vi "MPS_main.vi"() -> ()   [LabVIEW 2021] (continued)
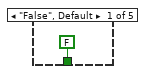
[diagram p2: hidden frame]
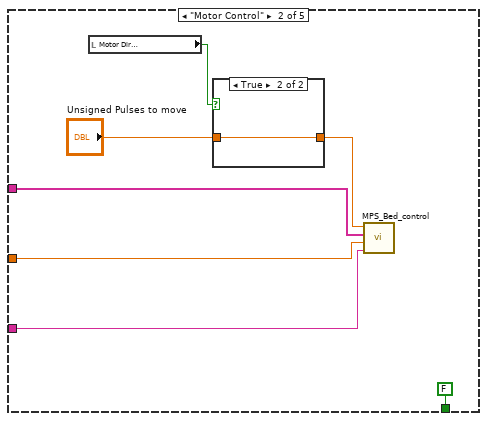
[diagram p3: hidden frame]
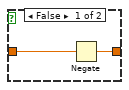
[diagram p4: hidden frame]
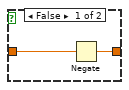
[diagram p5: hidden frame]
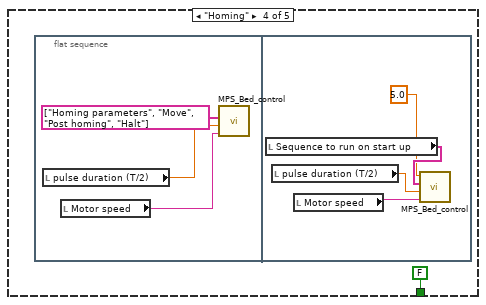
[diagram p6: hidden frame]
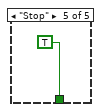
[diagram p7: hidden frame]
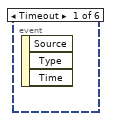
[diagram p8: hidden frame]
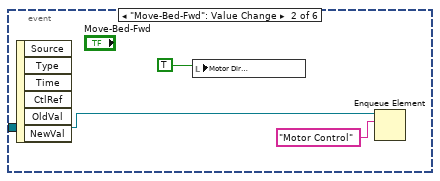
[diagram p9: hidden frame]
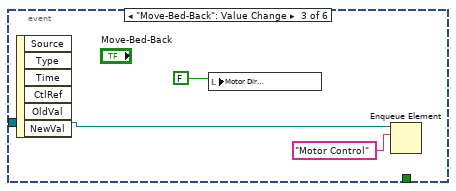
[diagram p10: hidden frame]
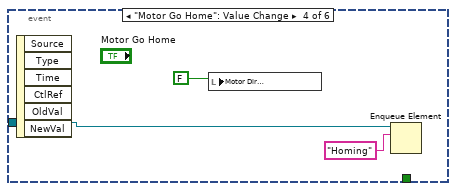
[diagram p11: hidden frame]
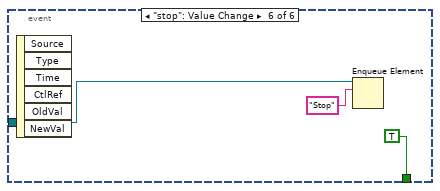
[diagram p12: hidden frame]
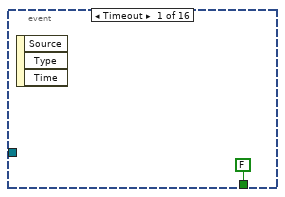
[diagram p13: hidden frame]
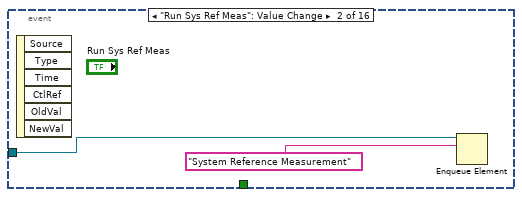
[diagram p14: hidden frame]
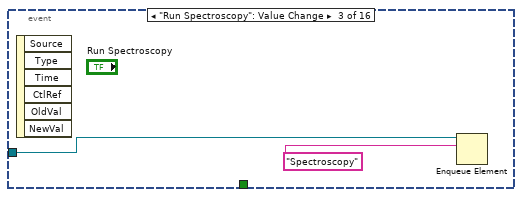
[diagram p15: hidden frame]
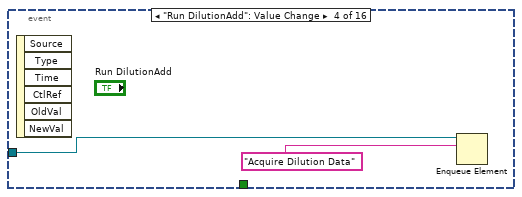
[diagram p16: hidden frame]
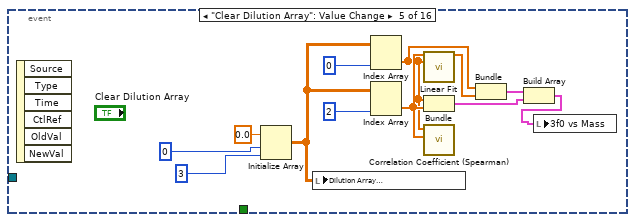
[diagram p17: hidden frame]
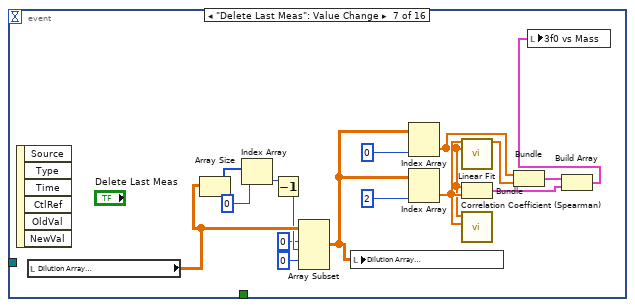
[diagram p18: hidden frame]
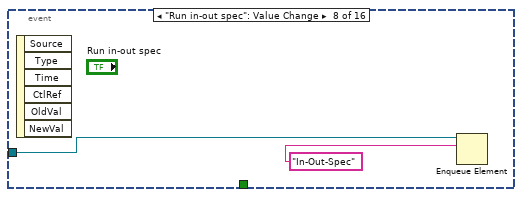
[diagram p19: hidden frame]
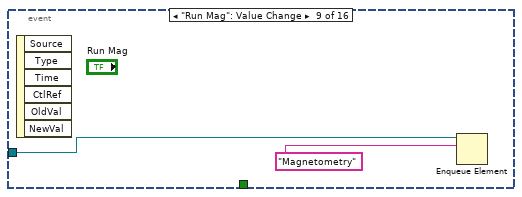
[diagram p20: hidden frame]
        n162 = Index Array(array=w205, index (col)=0 ("disabled index (col)")) -> (element=w206:dbl[])  [unwired: 1 in]
        n163 = call <vilib>:"Std Deviation and Variance.vi"("X"=w212) -> ("mean"=→"mean3f0":dbl, "standard deviation"=→"standard deviation 3f0":dbl)  [unwired: 1 in, 1 out]
        n164 = call <vilib>:"Std Deviation and Variance.vi"("X"=w206) -> ("mean"=→"meanf0":dbl, "standard deviation"=→"standard deviation f0":dbl)  [unwired: 1 in, 1 out]
        n165 = local read "Pulses From Home to Max Sig"() -> (w199:dbl)
        n166 = case shown="True" "Save Spectroscopy" {
          tunnel: w225 -> [_ w253]
          tunnel: w224 -> [_ w252]
          tunnel: w205 -> [_ w248]
          tunnel: w215 -> [_ w247]
          tunnel: w214 -> [_ w246]
          tunnel: w213 -> [_ w245]
          tunnel: w203 -> [_ w244]
          tunnel: w202 -> [_ w243]
          tunnel: w201 -> [_ w242]
          tunnel: w200 -> [_ w240]
          tunnel: w199 -> [_ w236]
          frame False {
          }
          frame True {
            w229 = u16 0 items=["Spec.", "Mag.", "In Out Spec"] ("Ring")
            n167 = local read "Sample MetaData Cluster"() -> (w230:T1)
            n168 = local read "name identifier"() -> (w231:string)
            n169 = local read "Study and Experiment Description"() -> (w234:T5)
            n170 = local read "Sample MetaData Cluster"() -> (w233:T1)
            n171 = Initialize Array(0.0 ("element"), 1 ("dimension size")) -> (w237:dbl[])
            n172 = local read "Base path"() -> (w232:path)
            n173 = call "Spectrometer_File_Naming.vi"("Description"=w231, "Sample MetaData Cluster"=w230, "Ring"=w229) -> ("Output Name"=w228:string)  [unwired: 8 in]
            n174 = Bundle By Name(cluster=T8 {"Drive IMon"=array[500000 elements], "Rx Time Domain"=array[500000 elements], "Rx Empty Bore"=array[500000 elements], "BMon"=array[500000 elements], "Bias IMon"=array[500000 elements], "TF-Corr-MagOverTime"=[], "Interpolated Rx TF-Mag"=[], "Interpolated Rx TF-Phase"=[]} ("Time Domain Cluster"), "Drive IMon"=w246, "Rx Time Domain"=w245, "Rx Empty Bore"=w253, "BMon"=w252, "Bias IMon"=w237, "TF-Corr-MagOverTime"=w244, "Interpolated Rx TF-Mag"=w243, "Interpolated Rx TF-Phase"=w240) -> (w254:T8)
            n175 = local read "Scanner Description"() -> (w235:T4)
            n176 = call "file_path.vi"("name identifier"=w228, "Base path"=w232) -> ("HDF path"=w250:path)  [unwired: 7 in, 2 out]
            n177 = global read "MPS_global_variables.vi" "TxRx_Params"() -> (w249:T2)
            n178 = local write "Recent File Name"(w228) -> ()
            n179 = call "save_MPS_spectroscopy_hdf.vi"("file path"=w250, "Device Name"=tag "H1", "Phase Rx over time"=w247, "Mag Rx over time"=w248, "TxRx_Params"=w249, "Rx_f0-f8 Units"=w242, "Time Domain Cluster"=w254, "Sample MetaData Cluster"=w233, "Study and Experiment Description"=w234, "Scanner Description"=w235, "Points from home to max"=w236) -> ()  [unwired: 5 in]
          }
        }
      }
      frame "Acquire Dilution Data" {
        n180 = Enqueue Element(queue=w325, element="Idle") -> ()  [unwired: 2 in, 3 out]
        n181 = Initialize Array(0.0 ("element"), 0 ("dimension size"), 9 ("dimension size")) -> (w322:dbl[][])
        n182 = while {
          shift-right: [w336] -> w317
          shift-left: w322 -> [w337]
          i -> [w335]
          stop <- w328 stop-if-true
          n183 = local read "RxEmptyBore-Spec"() -> (w334:dbl[])
          n184 = call "MPS_Spectroscopy_Core.vi"("EmptyBoreBaseline_Spec"=w334, "ms delay"="ms delay 2", "Spec samples\nto crop"="Spec samples\nto crop 3") -> ("mag f1-f9"=w331:dbl[], "Expected mT Spec Drive"=→"Expected mT Spec Drive 3":dbl, "THD"=→"THD 2":dbl)  [unwired: 2 in, 12 out]
          n185 = Insert Into Array(array=w337, index (row)=w335, new element=w331) -> (w336:dbl[][])  [unwired: 1 in]
          n186 = Greater Or Equal?(x=w335, y="Num Dil Series Runs") -> (x >= y?=w328:bool)
        }
        n187 = local read "Dilution Array\nConc,f0,f3"() -> (w315:dbl[][])
        n188 = local read "Sample MetaData Cluster"() -> (w310:T1)
        n189 = Index Array(array=w317, index (col)=2 ("index")) -> (element=w320:dbl[])  [unwired: 1 in]
        n190 = Index Array(array=w317, index (col)=0 ("disabled index (col)")) -> (element=w318:dbl[])  [unwired: 1 in]
        n191 = call <vilib>:"Std Deviation and Variance.vi"("X"=w318) -> ("mean"=w302:dbl)  [unwired: 1 in, 2 out]
        n192 = call <vilib>:"Std Deviation and Variance.vi"("X"=w320) -> ("mean"=w303:dbl)  [unwired: 1 in, 2 out]
        n193 = Unbundle By Name(w310) -> ("Sample Mass (ug)"=w311:dbl)
        n194 = Array Size(array=w315) -> (size(s)=w314:i32[])
        n195 = Index Array(array=w314, index=0) -> (element=w313:i32)
        n196 = Build Array(w311, w302, w303) -> (w309:dbl[])
        n197 = Bundle By Name(cluster=T9 {"slope min"=-inf, "slope max"=inf, "intercept min"=-inf, "intercept max"=inf} ("parameter bounds"), "intercept min"=0.0) -> (w295:T9)
        n198 = Insert Into Array(array=w315, index (row)=w313, new element=w309) -> (w307:dbl[][])  [unwired: 1 in]
        n199 = local write "Dilution Array\nConc,f0,f3"(w307) -> ()
        n200 = Index Array(array=w307, index (col)=0 ("disabled index (col)")) -> (element=w301:dbl[])  [unwired: 1 in]
        n201 = Index Array(array=w307, index (col)=2 ("disabled index (col)")) -> (element=w299:dbl[])  [unwired: 1 in]
        n202 = call <vilib>:"Linear Fit.vi"("Y"=w299, "X"=w301, "parameter bounds"=w295) -> ("Best Linear Fit"=w305:dbl[])  [unwired: 8 in, 4 out]
        n203 = call <vilib>:"Correlation Coefficient.vi"("Y"=w299, "X"=w301) -> ("r^2"=→"r^2":dbl)  [unwired: 8 in, 1 out]
        n204 = Bundle("Dilution Array\nConc,f0,f3"=w301, "Dilution Array\nConc,f0,f3"=w299) -> (w298:T13)  [unwired: 1 in]
        n205 = Bundle("Dilution Array\nConc,f0,f3"=w301, "Best Linear Fit"=w305) -> (w297:T14)  [unwired: 1 in]
        n206 = Build Array(w297, w298) -> (→"3f0 vs Mass":T6)
      }
      frame "In-Out-Spec" {
        w375 = 0
        n207 = Enqueue Element(queue=w393, element="Idle") -> ()  [unwired: 2 in, 3 out]
        n208 = Initialize Array(0.0 ("element"), 9 ("dimension size"), 1 ("dimension size")) -> (w376:dbl[][])
        n209 = Initialize Array(0.0 ("element"), 9 ("dimension size"), 1 ("dimension size")) -> (w377:dbl[][])
        n210 = Initialize Array(0.0 ("element"), 1 ("dimension size")) -> (w361:dbl[])
        n211 = Multiply(x="Number of cycles", y=2) -> (x*y=w365:i32)
        n212 = flat-sequence {
          tunnel: w377 -> [w404]
          tunnel: w376 -> [w403]
          tunnel: w375 -> [w402]
          tunnel: w365 -> [w399]
          tunnel: w361 -> [w398]
          tunnel: cluster{"f0":dbl, "df":dbl, "magnitude":dbl[]} {"f0"=0.0, "df"=49.55401387512537, "magnitude"=array[10090 elements]} ("Rx FFT 3") -> [w396]
          tunnel: [w401] -> w350
          tunnel: [w400] -> w349
          tunnel: [w397] -> w348
          tunnel: [w395] -> w347
          tunnel: [w498] -> w355
          tunnel: [w499] -> w360
          tunnel: [w500] -> w370
          tunnel: [w501] -> w374
          tunnel: w350 -> [w501]
          tunnel: w349 -> [w500]
          tunnel: w348 -> [w499]
          tunnel: w347 -> [w498]
          tunnel: [w495] -> w346
          tunnel: [w494] -> w345
          tunnel: [w493] -> w344
          frame #0 {
            n213 = for {
              N: w399 -> [_]
              shift-right: [w421] -> w400
              shift-left: w404 -> [w423]
              shift-right: [w420] -> w401
              shift-left: w403 -> [w422]
              tunnel: w402 -> [_]
              shift-right: [w411] -> w397
              shift-left: w398 -> [w412]
              shift-right: [w405] -> w395
              shift-left: w396 -> [_]
              i -> [w419]
              n214 = flat-sequence {
                tunnel: w423 -> [w433]
                tunnel: w422 -> [w432]
                tunnel: [w431] -> w416
                tunnel: [w430] -> w415
                tunnel: w414 -> [w429]
                tunnel: w412 -> [w428]
                tunnel: w407 -> [w427]
                tunnel: [w426] -> w410
                tunnel: [w425] -> w406
                tunnel: [w424] -> w405
                tunnel: [w488] -> w420
                tunnel: [w489] -> w421
                tunnel: w416 -> [w489]
                tunnel: w415 -> [w488]
                tunnel: w413 -> [w483]
                tunnel: [w473] -> w411
                tunnel: w410 -> [w473]
                tunnel: w406 -> [_]
                frame #0 {
                  n215 = while {
                    shift-right: [w470] -> w431
                    shift-left: w433 -> [w471]
                    shift-right: [w465] -> w430
                    shift-left: w432 -> [w469]
                    tunnel: w429 -> [w447]
                    tunnel: w427 -> [w441]
                    shift-right: [w440] -> w426
                    shift-left: w428 -> [w443]
                    tunnel: [w436] -> w425
                    tunnel: [w435] -> w424
                    i -> [w450]
                    stop <- w466 stop-if-true
                    w459 = T11 1 items=["Rectangle"=0, "Hanning"=1, "Hamming"=2, "Blackman-Harris"=3, "Exact Blackman"=4, "Blackman"=5, "Flat Top"=6, "4 Term B-Harris "=7, "7 Term B-Harris"=8, "Low Sidelobe"=9, "Blackman Nuttall"=11, "Triangle"=30, "Bartlett-Hanning"=31, "Bohman"=32, "Parzen"=33, "Welch"=34, "Kaiser"=60, "Dolph-Chebyshev"=61, "Gaussian"=62] ("window")
                    n216 = local read "RxEmptyBore-Spec"() -> (w464:dbl[])
                    n217 = local write "Bed moving"(FALSE ("Bed moving")) -> ()
                    n218 = local read "Run number"() -> (w451:i32)
                    n219 = Greater Or Equal?(x=w450, y="Num acq per\ncycle") -> (x >= y?=w466:bool)
                    n220 = Increment(x=w451) -> (x+1=w442:i32)
                    n221 = call "MPS_Spectroscopy_Core.vi"("EmptyBoreBaseline_Spec"=w464, "ms delay"="ms delay\nevery Spec", "Spec samples\nto crop"="Spec samples\nto crop_InOut") -> ("Raw Measured"=w444:dbl[], "f0 Complex"=w454:cdb, "phase f1-f9"=w467:dbl[], "TF Corr Rx FFT Mag"=→"Rx FFT 2":cluster{"f0":dbl, "df":dbl, "magnitude":dbl[]}, "Spec Waveform Baseline Sub"=w458:waveform(dbl), "3f0 Complex"=w457:cdb, "mag f1-f9"=w452:dbl[], "Expected mT Spec Drive"=→"Expected mT Spec Drive 2":dbl, "TF Corrected\nMagnetization over time"=w439:waveform(dbl)[], "Spec Time Domain"=→"Spec Time Domain 2":dbl[][], "THD"=→"Drive Imon THD 2":dbl)  [unwired: 2 in, 4 out]
                    n222 = Equal?(x=w450, y=0) -> (x = y?=w446:bool)
                    n223 = local write "Run number"(w442) -> ()
                    n224 = And(x=w446, y=w447) -> (x .and. y?=w448:bool)
                    n225 = Insert Into Array(array=w471, index (col)=w442, new element=w452) -> (w470:dbl[][])  [unwired: 1 in]
                    n226 = Insert Into Array(array=w469, index (col)=w442, new element=w467) -> (w465:dbl[][])  [unwired: 1 in]
                    n227 = Complex To Polar(r * e^(i*theta)=w454) -> (r=→"f0 over time 2":dbl)  [unwired: 1 out]
                    n228 = Complex To Polar(r * e^(i*theta)=w457) -> (r=→"3f0 over time 2":dbl)  [unwired: 1 out]
                    n229 = case shown="True" w448 {
                      tunnel: w444 -> [_ w472]
                      frame False {
                      }
                      frame True {
                        n230 = local write "RxEmptyBore-Spec"(w472) -> ()
                      }
                    }
                    n231 = Insert Into Array(array=w443, index=w442, new element=w441) -> (w440:dbl[])
                    n232 = Index Array(array=w439, index=1) -> (element=w437:waveform(dbl))
                    n233 = call-poly <vilib>:"FFT Spectrum (Mag-Phase).vi"("window"=w459, "time signal"=w458) -> ("magnitude"=w435:cluster{"f0":dbl, "df":dbl, "magnitude":dbl[]})  [unwired: 5 in, 4 out]
                    n234 = Unbundle By Name(w437) -> ("Y"=w436:dbl[])
                    "Loop Num 2" <- w450
                  }
                }
                frame #1 {
                  w480 = 0.0005 ("pulse duration (T/2)")
                  n235 = case shown="True" w483 {
                    tunnel: [w490 w491] -> w487
                    tunnel: "Pulses in/out" -> [w490 w492]
                    frame False {
                    }
                    frame True {
                      n236 = Negate(x=w492) -> (-x=w491:dbl)
                    }
                  }
                  n237 = local write "Bed moving"(TRUE) -> ()
                  n238 = Multiply(x="Pulses in/out", y=w480) -> (x*y=w482:dbl)
                  n239 = Multiply(x=w482, y=16.0) -> (x*y=w479:dbl)
                  n240 = Multiply(x=w479, y=1.25) -> (x*y=w477:dbl)
                  n241 = call "MPS_Bed_control.vi"("Motor speed"="Sixteenth step", "pulse duration (T/2)"=w480, "Sequence to run on start up"=string[] ["Move", "Halt"] ("Sequence to run on start up\n 2"), "Signed pulses to move"=w487) -> ()  [unwired: 8 in]
                  n242 = Multiply(x=1000.0, y=w477) -> (x*y=w475:dbl)
                  n243 = Wait (ms)(milliseconds to wait=w475) -> ()  [unwired: 1 out]
                }
              }
              n244 = Quotient & Remainder(x=w419, y=2) -> (x-y*floor(x/y)=w409:i32)  [unwired: 1 out]
              n245 = Decrement(x=w409) -> (x-1=w408:i32)
              n246 = Equal?(x=w409, y=0) -> (x = y?=w413:bool)
              n247 = Absolute Value(x=w408) -> (abs(x)=w407:i32)
              n248 = Not(x=w413) -> (.not. x?=w414:bool)
            }
          }
          frame #1 {
            # "Final Acq.\nwith sample in\nto save time domain"
            n249 = local read "Spec samples\nto crop_InOut"() -> (w496:dbl)
            n250 = local read "RxEmptyBore-Spec"() -> (w497:dbl[])
            n251 = call "MPS_Spectroscopy_Core.vi"("EmptyBoreBaseline_Spec"=w497, "Spec samples\nto crop"=w496) -> ("Spec Waveform Baseline Sub"=w495:waveform(dbl), "Drive IMon"=w494:waveform(dbl), "TF Corrected\nMagnetization over time"=w493:waveform(dbl)[])  [unwired: 3 in, 12 out]
          }
        }
        n252 = Unbundle By Name(w346) -> ("Y"=w341:dbl[])
        n253 = Unbundle By Name(w345) -> ("Y"=w340:dbl[])
        n254 = Array Subset(array=w370, index (row)=0 ("index"), index (col)=1 ("index")) -> (w369:dbl[][])  [unwired: 2 in]
        n255 = Array Subset(array=w374, index (row)=0 ("index"), index (col)=1 ("index")) -> (w373:dbl[][])  [unwired: 2 in]
        n256 = Array Subset(array=w360, index=1) -> (w358:dbl[])  [unwired: 1 in]
        n257 = Index Array(array=w344, index=1) -> (element=w342:waveform(dbl))
        n258 = Unbundle By Name(w342) -> ("Y"=w339:dbl[])
        n259 = local read "Study and Experiment Description"() -> (w386:T5)
        n260 = local read "Sample MetaData Cluster"() -> (w385:T1)
        n261 = local read "Empty Bore-BMon-Spec"() -> (w389:dbl[])
        n262 = global read "MPS_global_variables.vi" "Rx TF File"() -> (w354:string)
        n263 = local read "Scanner Description"() -> (w387:T4)
        n264 = local read "RxEmptyBore-Spec"() -> (w388:dbl[])
        n265 = call "get_freq_vector.vi"("FFT magnitude"=w355) -> ("Freq array"=w357:dbl[])  [unwired: 10 in]
        n266 = call "loadTF_resample.vi"("desired freqs"=w357, "mat file name"=w354) -> ("TF units from loaded file"=w351:string, "output TF phase"=w352:dbl[], "output TF mag"=w353:dbl[])  [unwired: 7 in]
        n267 = Initialize Array(0.0 ("element"), 1 ("dimension size")) -> (w390:dbl[])
        n268 = local read "Pulses From Home to Max Sig"() -> (w338:dbl)
        n269 = case shown="True" "Save Spectroscopy 2" {
          tunnel: w388 -> [_ w527]
          tunnel: w389 -> [_ w526]
          tunnel: w385 -> [_ w525]
          tunnel: w386 -> [_ w524]
          tunnel: w387 -> [_ w523]
          tunnel: w390 -> [_ w516]
          tunnel: w369 -> [_ w518]
          tunnel: w373 -> [_ w519]
          tunnel: w358 -> [_ w517]
          tunnel: w353 -> [_ w515]
          tunnel: w352 -> [_ w513]
          tunnel: w351 -> [_ w512]
          tunnel: w341 -> [_ w511]
          tunnel: w340 -> [_ w510]
          tunnel: w339 -> [_ w509]
          tunnel: w338 -> [_ w507]
          frame False {
          }
          frame True {
            w503 = u16 2 items=["Spec.", "Mag.", "In Out Spec"] ("Ring")
            n270 = local read "Sample MetaData Cluster"() -> (w505:T1)
            n271 = Bundle By Name(cluster=T8 {"Drive IMon"=array[500000 elements], "Rx Time Domain"=array[500000 elements], "Rx Empty Bore"=array[500000 elements], "BMon"=array[500000 elements], "Bias IMon"=array[500000 elements], "TF-Corr-MagOverTime"=[], "Interpolated Rx TF-Mag"=[], "Interpolated Rx TF-Phase"=[]} ("Time Domain Cluster 2"), "Drive IMon"=w510, "Rx Time Domain"=w511, "Rx Empty Bore"=w527, "BMon"=w526, "Bias IMon"=w516, "TF-Corr-MagOverTime"=w509, "Interpolated Rx TF-Mag"=w515, "Interpolated Rx TF-Phase"=w513) -> (w508:T8)
            n272 = local read "Base path"() -> (w504:path)
            n273 = local read "name identifier"() -> (w506:string)
            n274 = call "Spectrometer_File_Naming.vi"("Description"=w506, "Sample MetaData Cluster"=w505, "Ring"=w503) -> ("Output Name"=w502:string)  [unwired: 8 in]
            n275 = global read "MPS_global_variables.vi" "TxRx_Params"() -> (w520:T2)
            n276 = call "file_path.vi"("name identifier"=w502, "Base path"=w504) -> ("HDF path"=w521:path)  [unwired: 7 in, 2 out]
            n277 = local write "Recent File Name"(w502) -> ()
            n278 = call "save_MPS_spectroscopy_hdf.vi"("file path"=w521, "Device Name"=tag "H1", "Phase Rx over time"=w519, "Mag Rx over time"=w518, "TxRx_Params"=w520, "Rx_f0-f8 Units"=w512, "Time Domain Cluster"=w508, "Sample MetaData Cluster"=w525, "Study and Experiment Description"=w524, "Sample in_vs_Out"=w517, "Scanner Description"=w523, "Points from home to max"=w507) -> ()  [unwired: 4 in]
          }
        }
        "Run number" <- w375
      }
      frame "Update Meta" {
      }
      frame "Magnetometry" {
        w551 = T11 1 items=["Rectangle"=0, "Hanning"=1, "Hamming"=2, "Blackman-Harris"=3, "Exact Blackman"=4, "Blackman"=5, "Flat Top"=6, "4 Term B-Harris "=7, "7 Term B-Harris"=8, "Low Sidelobe"=9, "Blackman Nuttall"=11, "Triangle"=30, "Bartlett-Hanning"=31, "Bohman"=32, "Parzen"=33, "Welch"=34, "Kaiser"=60, "Dolph-Chebyshev"=61, "Gaussian"=62] ("window")
        n279 = Enqueue Element(queue=w560, element="Idle") -> ()  [unwired: 2 in, 3 out]
        n280 = local read "EmptyBoreBaseline_Mag"() -> (w542:dbl[])
        n281 = Array Size(array=w542) -> (size(s)=w538:i32)
        n282 = Initialize Array(0.0 ("element"), w538) -> (w537:dbl[])
        n283 = Initialize Array(0.0 ("element"), w538, "Num Mag Avgs") -> (w543:dbl[][])
        n284 = Multiply(x="Num Mag Avgs", y=2) -> (x*y=w532:i32)
        n285 = for {
          N: w532 -> [_]
          tunnel: [w582] -> w530
          tunnel: [w581] -> w552
          tunnel: [w580] -> w535
          shift-right: [w578] -> w540
          shift-left: w543 -> [w579]
          i -> [w572]
          n286 = Quotient & Remainder(x=w572, y=2) -> (x-y*floor(x/y)=w575:i32, floor(x/y)=w571:i32)
          n287 = flat-sequence {
            tunnel: [w597] -> w582
            tunnel: [w584] -> w580
            tunnel: w579 -> [w590]
            tunnel: [w595] -> w577
            tunnel: [w588] -> w576
            tunnel: w567 -> [w591]
            tunnel: w571 -> [w587]
            tunnel: w577 -> [w622]
            tunnel: w576 -> [w621]
            tunnel: w570 -> [w613]
            tunnel: [w622] -> w569
            tunnel: [w621] -> w568
            tunnel: [w627] -> w578
            tunnel: [w628] -> w581
            tunnel: w569 -> [w628]
            tunnel: w568 -> [w627]
            frame #0 {
              n288 = local read "EmptyBoreBaseline_Mag_BMon"() -> (w599:dbl[])
              n289 = local read "EmptyBoreBaseline_Mag"() -> (w600:dbl[])
              n290 = local write "Bed moving"(FALSE) -> ()
              n291 = call "MPS_Mag_Core.vi"("EmptyBoreBaseline_Mag_BMon"=w599, "EmptyBoreBaseline_Mag"=w600) -> ("Samples Per Acquisition"=w593:dbl, "Drive IMon"=w596:waveform(dbl), "Susceptibility Curves"=→"Susceptibility Curves":cluster{"Y":dbl[], "Y":dbl[]}[], "Rx Smooth"=→"Rx Smooth":dbl[], "Bias Current"=w597:waveform(dbl), "Rx_Raw"=w585:waveform(dbl), "RxBaselineSub"=w584:waveform(dbl))  [unwired: 5 in, 2 out]
              n292 = local write "Samples Per Acquisition"(w593) -> ()
              n293 = Unbundle By Name(w596) -> ("Y"=w595:dbl[])
              n294 = call "MPS_Mag_Proc_Spectrogram.vi"("Signal"=w584) -> ("Sensitivity profile"=→"Sensitivity profile":dbl[][])  [unwired: 9 in, 1 out]
              n295 = Unbundle By Name(w584) -> ("Y"=w583:dbl[])
              n296 = Unbundle By Name(w585) -> ("Y"=w589:dbl[])
              n297 = case shown="False" w591 {
                tunnel: w590 -> [w604 w606]
                tunnel: w589 -> [_ w605]
                tunnel: [w603 w606] -> w588
                tunnel: w587 -> [w602 _]
                tunnel: w583 -> [w601 _]
                frame False {
                  n298 = Replace Array Subset(array=w604, new element=w601, index (col)=w602) -> (w603:dbl[][])  [unwired: 1 in]
                  "RunNum" <- w602
                }
                frame True {
                  n299 = local write "EmptyBoreBaseline_Mag"(w605) -> ()
                }
              }
            }
            frame #1 {
              w611 = 0.0005 ("pulse duration (T/2)")
              n300 = case shown="True" w613 {
                tunnel: [w623 w624] -> w615
                tunnel: "Pulses in/out 2" -> [w623 w625]
                frame False {
                }
                frame True {
                  n301 = Negate(x=w625) -> (-x=w624:dbl)
                }
              }
              n302 = local write "Bed moving"(TRUE) -> ()
              n303 = Multiply(x="Pulses in/out 2", y=w611) -> (x*y=w616:dbl)
              n304 = Multiply(x=w616, y=16.0) -> (x*y=w617:dbl)
              n305 = Multiply(x=w617, y=1.25) -> (x*y=w618:dbl)
              n306 = call "MPS_Bed_control.vi"("Motor speed"="Sixteenth step", "pulse duration (T/2)"=w611, "Sequence to run on start up"=string[] ["Move", "Halt"] ("Sequence to run on start up\n 2"), "Signed pulses to move"=w615) -> ()  [unwired: 8 in]
              n307 = Multiply(x=1000.0, y=w618) -> (x*y=w619:dbl)
              n308 = Wait (ms)(milliseconds to wait=w619) -> ()  [unwired: 1 out]
            }
            frame #2 {
              n309 = Wait (ms)(milliseconds to wait="ms delay each run") -> ()  [unwired: 1 out]
            }
          }
          n310 = Equal?(x=w575, y=0) -> (x = y?=w570:bool)
          n311 = Not(x=w570) -> (.not. x?=w567:bool)
          "Sample Out" <- w567
          "Numeric" <- w572
        }
        n312 = for {
          N: "Num Mag Avgs" -> [_]
          shift-right: [w563] -> w536
          shift-left: w537 -> [w564]
          shift-right: [w562] -> _
          shift-left: w540 -> [w562]
          i -> [w566]
          n313 = Index Array(array=w562, index (col)=w566) -> (element=w565:dbl[])  [unwired: 1 in]
          n314 = Add(x=w565, y=w564) -> (x+y=w563:dbl[])
        }
        n315 = call-poly <vilib>:"FFT Spectrum (Mag-Phase).vi"("window"=w551, "time signal"=w535) -> ("magnitude"=w549:cluster{"f0":dbl, "df":dbl, "magnitude":dbl[]})  [unwired: 5 in, 4 out]
        n316 = global read "MPS_global_variables.vi" "Rx TF File"() -> (w548:string)
        n317 = Unbundle By Name(w530) -> ("Y"=w553:dbl[])
        n318 = call "get_freq_vector.vi"("FFT magnitude"=w549) -> ("Freq array"=w550:dbl[])  [unwired: 10 in]
        n319 = call "loadTF_resample.vi"("desired freqs"=w550, "mat file name"=w548) -> ("TF units from loaded file"=w545:string, "output TF phase"=w547:dbl[], "output TF mag"=w546:dbl[])  [unwired: 7 in]
        n320 = local read "Study and Experiment Description"() -> (w556:T5)
        n321 = local read "EmptyBoreBaseline_Mag_BMon"() -> (w558:dbl[])
        n322 = Divide(x=w536, y="Num Mag Avgs") -> (x/y=w531:dbl[])
        n323 = local read "Sample MetaData Cluster"() -> (w557:T1)
        n324 = local read "Scanner Description"() -> (w555:T4)
        n325 = local read "EmptyBoreBaseline_Mag"() -> (w559:dbl[])
        n326 = Bundle By Name(cluster=w530, "Y"=w531) -> (w529:waveform(dbl))
        n327 = call "MPS_Mag_Proc_Spectrogram.vi"("Signal"=w529) -> ("Sensitivity profile"=→"Sensitivity profile 2":dbl[][])  [unwired: 9 in, 1 out]
        n328 = local read "Pulses From Home to Max Sig"() -> (w544:dbl)
        n329 = case shown="True" "Save Mag data" {
          tunnel: w558 -> [_ w653]
          tunnel: w557 -> [_ w652]
          tunnel: w556 -> [_ w651]
          tunnel: w555 -> [_ w650]
          tunnel: w559 -> [_ w647]
          tunnel: w553 -> [_ w643]
          tunnel: w552 -> [_ w642]
          tunnel: w547 -> [_ w640]
          tunnel: w546 -> [_ w639]
          tunnel: w545 -> [_ w638]
          tunnel: w544 -> [_ w635]
          tunnel: w531 -> [_ w629]
          frame False {
          }
          frame True {
            w632 = u16 1 items=["Spec.", "Mag.", "In Out Spec"] ("Ring")
            n330 = local read "Sample MetaData Cluster"() -> (w634:T1)
            n331 = Bundle By Name(cluster=T8 {"Drive IMon"=array[500000 elements], "Rx Time Domain"=array[500000 elements], "Rx Empty Bore"=array[500000 elements], "BMon"=array[500000 elements], "Bias IMon"=array[500000 elements], "TF-Corr-MagOverTime"=[], "Interpolated Rx TF-Mag"=[], "Interpolated Rx TF-Phase"=[]} ("Time Domain Cluster 3"), "Drive IMon"=w642, "Rx Time Domain"=w629, "Rx Empty Bore"=w647, "BMon"=w653, "Bias IMon"=w643, "TF-Corr-MagOverTime"=dbl[] [], "Interpolated Rx TF-Mag"=w639, "Interpolated Rx TF-Phase"=w640) -> (w637:T8)
            n332 = local read "name identifier"() -> (w633:string)
            n333 = local read "Base path"() -> (w631:path)
            n334 = call "Spectrometer_File_Naming.vi"("Description"=w633, "Sample MetaData Cluster"=w634, "Ring"=w632) -> ("Output Name"=w630:string)  [unwired: 8 in]
            n335 = global read "MPS_global_variables.vi" "TxRx_Params"() -> (w645:T2)
            n336 = call "file_path.vi"("name identifier"=w630, "Base path"=w631) -> ("HDF path"=w648:path)  [unwired: 7 in, 2 out]
            n337 = Initialize Array(0.0 ("element")) -> (w644:dbl[][])  [unwired: 2 in]
            n338 = call "save_MPS_spectroscopy_hdf.vi"("file path"=w648, "Device Name"=tag "H1", "Phase Rx over time"=w644, "Mag Rx over time"=w644, "TxRx_Params"=w645, "Rx_f0-f8 Units"=w638, "Time Domain Cluster"=w637, "Sample MetaData Cluster"=w652, "Study and Experiment Description"=w651, "Scanner Description"=w650, "Points from home to max"=w635) -> ()  [unwired: 5 in]
            n339 = local write "Recent File Name"(w630) -> ()
          }
        }
      }
      frame "Acquire Empty Bore" {
        n340 = Enqueue Element(queue=w654, element="Idle") -> ()  [unwired: 2 in, 3 out]
        n341 = stacked-sequence {
          frame #0 {
            # "Data queue"
            # "Data queue"
            n342 = global read "MPS_global_variables.vi" "TxRx_Params"() -> (w665:T2)
            n343 = Unbundle By Name(w665) -> ("Tx cycles\nSpectroscopy"=w661:dbl, "sample rate"=w664:dbl, "Tx freq"=w663:dbl)
            n344 = Obtain Queue(element data type=waveform(dbl) {"t0"=timestamp(0 s since 1904-01-01), "dt"=1.0, "Y"=[]} ("Waveform")) -> (queue out=w666:refnum<queue>)  [unwired: 4 in, 2 out]
            n345 = Obtain Queue(element data type=waveform(dbl) {"t0"=timestamp(0 s since 1904-01-01), "dt"=1.0, "Y"=[]} ("Waveform")) -> (queue out=w658:refnum<queue>)  [unwired: 4 in, 2 out]
            n346 = Divide(x=w664, y=w663) -> (x/y=w662:dbl)
            n347 = Multiply(x=w661, y=w662) -> (x*y=w660:dbl)
            n348 = flat-sequence {
              tunnel: w666 -> [w668]
              tunnel: w660 -> [w671]
              tunnel: [w670] -> w659
              tunnel: w659 -> [w691]
              tunnel: w658 -> [w678]
              frame #0 {
                w673 = T11 1 items=["Rectangle"=0, "Hanning"=1, "Hamming"=2, "Blackman-Harris"=3, "Exact Blackman"=4, "Blackman"=5, "Flat Top"=6, "4 Term B-Harris "=7, "7 Term B-Harris"=8, "Low Sidelobe"=9, "Blackman Nuttall"=11, "Triangle"=30, "Bartlett-Hanning"=31, "Bohman"=32, "Parzen"=33, "Welch"=34, "Kaiser"=60, "Dolph-Chebyshev"=61, "Gaussian"=62] ("window")
                n349 = call <extravilib>:"Write.vi"("element"=1 ("number of readouts")) -> ("channel"=w676:T12)  [unwired: 1 out]
                n350 = Dequeue Element(queue=w668) -> (element=w667:waveform(dbl))  [unwired: 2 in, 3 out]
                n351 = Round To Nearest(number=w671) -> (nearest integer value=w670:dbl)
                n352 = Unbundle By Name(w667) -> ("Y"=w674:dbl[])
                "EmptyBoreBaseline_Spec" <- w674
                "RxEmptyBore-Spec" <- w674
                n353 = call-poly <vilib>:"FFT Spectrum (Mag-Phase).vi"("window"=w673, "time signal"=w667) -> ("magnitude"=w672:cluster{"f0":dbl, "df":dbl, "magnitude":dbl[]})  [unwired: 5 in, 4 out]
                n354 = call "MPS_transmit_receive.vi"("samples per readout"=w670, "Use Bias?"=FALSE, "InputChans"=enum16{"Rx", "BiasIMon", "TxIMon", "BMon"}."Rx", "channel input for max readouts"=w676, "Measurement Queue"=w668) -> ()  [unwired: 7 in]
                n355 = local write "Samples Per Acquisition"(w670) -> ()
                n356 = local write "EmptyBoreBaseline_Spec"(w674) -> ()
                n357 = Complex To Polar(r * e^(i*theta)=w672) -> ()  [unwired: 2 out]
              }
              frame #1 {
                n358 = Dequeue Element(queue=w678) -> (element=w680:waveform(dbl))  [unwired: 2 in, 3 out]
                n359 = Round To Nearest(number=w691) -> (nearest integer value=w694:dbl)
                n360 = call <extravilib>:"Write.vi"("element"=1 ("number of readouts")) -> ("channel"=w695:T12)  [unwired: 1 out]
                n361 = call "MPS_transmit_receive.vi"("samples per readout"=w694, "Use Bias?"=TRUE, "InputChans"=enum16{"Rx", "BiasIMon", "TxIMon", "BMon"}."BMon", "channel input for max readouts"=w695, "Measurement Queue"=w678) -> ()  [unwired: 7 in]
                n362 = call-poly <vilib>:"Mean.vi"("X"=w680) -> ("mean"=w690:dbl)  [unwired: 1 out]
                n363 = Subtract(x=w680, y=w690) -> (x-y=w688:waveform(dbl))
                n364 = Unbundle By Name(w680) -> ("Y"=→"Empty Bore-BMon-Spec":dbl[], "dt"=w687:dbl)
                n365 = call <vilib>:"Integral x(t).vi"("dt"=w687, "Initial Condition"=dbl[] [0.0], "X"=w688) -> ("Integral X"=w686:dbl[])  [unwired: 7 in, 1 out]
                n366 = Bundle By Name(cluster=w680, "Y"=w686) -> (w682:waveform(dbl))
                n367 = call-poly <vilib>:"Extract Single Tone Information.vi"("export mode"=T10."detected signal", "time signal in"=w682) -> ("exported signals"=w684:T15)  [unwired: 4 in, 5 out]
                n368 = Unbundle By Name(w684) -> ("exported time signal"=w683:waveform(dbl))
                n369 = Unbundle By Name(w683) -> ()  [unwired: 1 out]
              }
            }
          }
          frame #1 {
            n370 = Wait (ms)(milliseconds to wait=u32 100) -> ()  [unwired: 1 out]
          }
          frame #2 {
            # "Data queue"
            # "Data queue"
            n371 = global read "MPS_global_variables.vi" "TxRx_Params"() -> (w706:T2)
            n372 = Unbundle By Name(w706) -> ("Bias Periods\nMagnetometry"=w702:dbl, "sample rate"=w705:dbl, "Bias freq"=w704:dbl)
            n373 = Obtain Queue(element data type=waveform(dbl) {"t0"=timestamp(0 s since 1904-01-01), "dt"=1.0, "Y"=[]} ("Waveform")) -> (queue out=w707:refnum<queue>)  [unwired: 4 in, 2 out]
            n374 = Obtain Queue(element data type=waveform(dbl) {"t0"=timestamp(0 s since 1904-01-01), "dt"=1.0, "Y"=[]} ("Waveform")) -> (queue out=w700:refnum<queue>)  [unwired: 4 in, 2 out]
            n375 = Divide(x=w705, y=w704) -> (x/y=w703:dbl)
            n376 = Multiply(x=w702, y=w703) -> (x*y=w701:dbl)
            n377 = flat-sequence {
              tunnel: w707 -> [w709]
              tunnel: w701 -> [w712]
              tunnel: [w712] -> w699
              tunnel: w700 -> [w718]
              tunnel: w699 -> [w720]
              frame #0 {
                n378 = Dequeue Element(queue=w709) -> (element=w710:waveform(dbl))  [unwired: 2 in, 3 out]
                "RxEmptyBore-Mag" <- w710
                n379 = Round To Nearest(number=w712) -> (nearest integer value=w714:dbl)
                n380 = call <extravilib>:"Write.vi"("element"=1 ("number of readouts")) -> ("channel"=w715:T12)  [unwired: 1 out]
                n381 = Unbundle By Name(w710) -> ("Y"=w711:dbl[])
                "EmptyBoreBaseline_Mag" <- w711
                n382 = call "MPS_transmit_receive.vi"("samples per readout"=w714, "Use Bias?"=TRUE, "InputChans"=enum16{"Rx", "BiasIMon", "TxIMon", "BMon"}."Rx", "channel input for max readouts"=w715, "Measurement Queue"=w709) -> ()  [unwired: 7 in]
                n383 = local write "Samples Per Acquisition"(w714) -> ()
                n384 = local write "EmptyBoreBaseline_Mag"(w711) -> ()
              }
              frame #1 {
                (unwired) FALSE ("T=DriveMon \nF=BMon")
                n385 = call <extravilib>:"Write.vi"("element"=1 ("number of readouts")) -> ("channel"=w722:T12)  [unwired: 1 out]
                n386 = Dequeue Element(queue=w718) -> (element=w719:waveform(dbl))  [unwired: 2 in, 3 out]
                n387 = Round To Nearest(number=w720) -> (nearest integer value=w723:dbl)
                n388 = Unbundle By Name(w719) -> ("Y"=w724:dbl[])
                "EmptyBoreBaseline_Mag_BMon" <- w724
                n389 = call "MPS_transmit_receive.vi"("samples per readout"=w723, "Use Bias?"=TRUE, "InputChans"=enum16{"Rx", "BiasIMon", "TxIMon", "BMon"}."BMon", "channel input for max readouts"=w722, "Measurement Queue"=w718) -> ()  [unwired: 7 in]
                n390 = local write "Samples Per Acquisition"(w723) -> ()
                n391 = local write "EmptyBoreBaseline_Mag_BMon"(w724) -> ()
              }
            }
          }
        }
      }
      frame "Halt" {
      }
    }
  }
  n392 = Format Date/Time String(time format string (%c)="%Y-%m-%d_%H-%m-%S") -> (date/time string=w4:string)  [unwired: 2 in]
  n393 = call <vilib>:"Create NI GUID.vi"() -> ("NI GUID"=w7:string)
  n394 = Bundle By Name(cluster="Study and Experiment Description", "UUID"=w7, "GUI Open Time"=w4) -> (w6:T5)
  n395 = Obtain Queue(name (unnamed)="Motor_Queue", element data type="") -> (queue out=w1:refnum<queue>)  [unwired: 3 in, 2 out]
  n396 = local write "Study and Experiment Description"(w6) -> ()
  n397 = while {
    tunnel: w1 -> [w728]
    stop <- w727 stop-if-true
    n398 = event shown="[4] \"Home then insert sample\": Value Change" {
      selector: _ -> [_ _ _ _ _ _]
      dyn-events: _ -> [_ _ _ _ _ _]
      timeout: _ -> [_ _ _ _ _ _]
      tunnel: w728 -> [_ w729 w732 w735 w740 w743]
      tunnel: [_ _ _ _ _ TRUE] -> w727
      event Timeout {
        n399 = event-data() -> ()  [unwired: 1 in, 3 out]
      }
      event "Move-Bed-Fwd": Value Change {
        n400 = event-data() -> ()  [unwired: 1 in, 6 out]
        n401 = local write "Motor Dir\nT=Fwd"(TRUE) -> ()
        n402 = Enqueue Element(queue=w729, element="Motor Control") -> ()  [unwired: 2 in, 3 out]
      }
      event "Move-Bed-Back": Value Change {
        n403 = event-data() -> ()  [unwired: 1 in, 6 out]
        n404 = local write "Motor Dir\nT=Fwd"(FALSE) -> ()
        n405 = Enqueue Element(queue=w732, element="Motor Control") -> ()  [unwired: 2 in, 3 out]
      }
      event "Motor Go Home": Value Change {
        n406 = event-data() -> ()  [unwired: 1 in, 6 out]
        n407 = local write "Motor Dir\nT=Fwd"(FALSE) -> ()
        n408 = Enqueue Element(queue=w735, element="Homing") -> ()  [unwired: 2 in, 3 out]
      }
      event "Home then insert sample": Value Change {
        n409 = event-data() -> ()  [unwired: 1 in, 6 out]
        n410 = local write "Motor Dir\nT=Fwd"(TRUE) -> ()
        n411 = Enqueue Element(queue=w740, element="Homing") -> (queue out=w738:refnum<queue>)  [unwired: 2 in, 2 out]
        n412 = Enqueue Element(queue=w738, element="MoveToMax") -> ()  [unwired: 2 in, 3 out]
      }
      event "stop": Value Change {
        n413 = event-data() -> ()  [unwired: 1 in, 6 out]
        n414 = Enqueue Element(queue=w743, element="Stop") -> ()  [unwired: 2 in, 3 out]
      }
    }
  }
  n415 = while {
    tunnel: w1 -> [w750]
    stop <- w749 stop-if-true
    n416 = Dequeue Element(queue=w750) -> (element=w751:string)  [unwired: 2 in, 3 out]
    "Current Motor State" <- w751
    n417 = case shown="\"MoveToMax\"" w751 {
      tunnel: [FALSE FALSE FALSE FALSE TRUE] -> w749
      tunnel: "Sequence to run on start up" -> [_ w755 w765 _ _]
      tunnel: "Motor speed" -> [_ w754 w763 _ _]
      tunnel: "pulse duration (T/2)" -> [_ w753 w764 _ _]
      frame "False", Default {
      }
      frame "Motor Control" {
        n418 = local read "Motor Dir\nT=Fwd"() -> (w757:bool)
        n419 = case shown="True" w757 {
          tunnel: [w760 w762] -> w758
          tunnel: "Unsigned Pulses to move" -> [w761 w762]
          frame False {
            n420 = Negate(x=w761) -> (-x=w760:dbl)
          }
          frame True {
          }
        }
        n421 = call "MPS_Bed_control.vi"("Motor speed"=w754, "pulse duration (T/2)"=w753, "Sequence to run on start up"=w755, "Signed pulses to move"=w758) -> ()  [unwired: 8 in]
      }
      frame "MoveToMax" {
        n422 = local read "Motor Dir\nT=Fwd"() -> (w768:bool)
        n423 = case shown="True" w768 {
          tunnel: [w770 w772] -> w769
          tunnel: "Pulses From Home to Max Sig" -> [w771 w772]
          frame False {
            n424 = Negate(x=w771) -> (-x=w770:dbl)
          }
          frame True {
          }
        }
        n425 = call "MPS_Bed_control.vi"("Motor speed"=w763, "pulse duration (T/2)"=w764, "Sequence to run on start up"=w765, "Signed pulses to move"=w769) -> ()  [unwired: 8 in]
      }
      frame "Homing" {
        n426 = flat-sequence {
          frame #0 {
            n427 = local read "pulse duration (T/2)"() -> (w775:dbl)
            n428 = local read "Motor speed"() -> (w774:string)
            n429 = call "MPS_Bed_control.vi"("Motor speed"=w774, "pulse duration (T/2)"=w775, "Sequence to run on start up"=string[] ["Homing parameters", "Move", "Post homing", "Halt"]) -> ()  [unwired: 9 in]
          }
          frame #1 {
            n430 = local read "Sequence to run on start up"() -> (w780:string[])
            n431 = local read "pulse duration (T/2)"() -> (w779:dbl)
            n432 = local read "Motor speed"() -> (w778:string)
            n433 = call "MPS_Bed_control.vi"("Motor speed"=w778, "pulse duration (T/2)"=w779, "Sequence to run on start up"=w780, "Signed pulses to move"=5.0) -> ()  [unwired: 8 in]
          }
        }
      }
      frame "Stop" {
      }
    }
  }
  n434 = local write "Main loop has stopped"(w12) -> ()
  "Main loop has stopped" <- FALSE ("Main loop has stopped")
